vi "Dresden R2R Sputter 03.02.2018 IY24.vi"() -> ()   [LabVIEW 2009] (continued)
                                }
                                }
                                }
                                }
                                frame #1 {
                                }
                                }
                                }
                                }
                              }
                              frame #17 {
                                # "CLOSE PC-BV"
                                n22872 = local read "Yes 4"() -> (w22132:bool)
                                n22873 = case shown="True" w22132 {
                                frame #0 {
                                }
                                frame #1 {
                                n22874 = local read "Semi"() -> (w22133:bool)
                                n22875 = case shown="False" w22133 {
                                frame #0 {
                                n22876 = stacked-sequence {
                                frame #0 {
                                n22877 = local read "Semi"() -> (w22134:bool)
                                n22878 = case shown="False" w22134 {
                                frame #0 {
                                n22879 = stacked-sequence {
                                frame #0 {
                                n22880 = local read "Semi"() -> (w22135:bool)
                                n22881 = case shown="False" w22135 {
                                frame #0 {
                                n22882 = local write "Pc_bv4_auto_close"(TRUE ("Tp1_auto_start")) -> ()
                                }
                                frame #1 {
                                }
                                }
                                }
                                frame #1 {
                                n22883 = local read "Semi"() -> (w22137:bool)
                                n22884 = case shown="False" w22137 {
                                frame #0 {
                                n22885 = Wait (ms)(milliseconds to wait=u32 1000) -> ()  [unwired: 1 out]
                                }
                                frame #1 {
                                }
                                }
                                }
                                frame #2 {
                                n22886 = local read "Semi"() -> (w22139:bool)
                                n22887 = case shown="False" w22139 {
                                frame #0 {
                                n22888 = while {
                                i -> [w22145]
                                stop <- w22141 stop-if-true
                                n22889 = local read "Pc_bv_closed_ch4"() -> (w22143:bool)
                                n22890 = Greater?(x=w22145, y=120) -> (0:w22144:bool)
                                n22891 = local read "Semi"() -> (w22142:bool)
                                n22892 = Compound Arithmetic op=OR(w22142, w22143, w22144) -> (w22141:bool)
                                n22893 = Wait (ms)(milliseconds to wait=u32 500) -> ()  [unwired: 1 out]
                                }
                                }
                                frame #1 {
                                }
                                }
                                }
                                frame #3 {
                                n22894 = local read "Semi"() -> (w22147:bool)
                                n22895 = case shown="False" w22147 {
                                frame #0 {
                                n22896 = local read "Pc_bv_closed_ch4"() -> (w22148:bool)
                                n22897 = case shown="False" w22148 {
                                frame #0 {
                                n22898 = local write "Pc_bv4_auto_close"(TRUE ("Pc_bv1_auto_open")) -> ()
                                }
                                frame #1 {
                                }
                                }
                                }
                                frame #1 {
                                }
                                }
                                }
                                frame #4 {
                                n22899 = local read "Semi"() -> (w22150:bool)
                                n22900 = case shown="False" w22150 {
                                frame #0 {
                                n22901 = local read "Pc_bv_closed_ch1"() -> (w22151:bool)
                                n22902 = case shown="False" w22151 {
                                frame #0 {
                                n22903 = Wait (ms)(milliseconds to wait=u32 1000) -> ()  [unwired: 1 out]
                                }
                                frame #1 {
                                }
                                }
                                }
                                frame #1 {
                                }
                                }
                                }
                                frame #5 {
                                n22904 = local read "Semi"() -> (w22153:bool)
                                n22905 = case shown="False" w22153 {
                                frame #0 {
                                n22906 = while {
                                i -> [w22159]
                                stop <- w22155 stop-if-true
                                n22907 = local read "Pc_bv_closed_ch4"() -> (w22157:bool)
                                n22908 = Greater?(x=w22159, y=120) -> (0:w22158:bool)
                                n22909 = local read "Semi"() -> (w22156:bool)
                                n22910 = Compound Arithmetic op=OR(w22156, w22157, w22158) -> (w22155:bool)
                                n22911 = Wait (ms)(milliseconds to wait=u32 500) -> ()  [unwired: 1 out]
                                }
                                }
                                frame #1 {
                                }
                                }
                                }
                                frame #6 {
                                n22912 = local read "Semi"() -> (w22161:bool)
                                n22913 = case shown="False" w22161 {
                                frame #0 {
                                n22914 = local read "Pc_bv_closed_ch4"() -> (w22162:bool)
                                n22915 = case shown="False" w22162 {
                                frame #0 {
                                n22916 = local write "Error Message"("Shut Down process  cancelled\nbecause  PC-BV not closed.\nPlease check PC-BV4 connections." ("Error Message")) -> ()
                                n22917 = Wait (ms)(milliseconds to wait=u32 1000) -> ()  [unwired: 1 out]
                                }
                                frame #1 {
                                }
                                }
                                }
                                frame #1 {
                                }
                                }
                                }
                                }
                                }
                                frame #1 {
                                }
                                }
                                }
                                frame #1 {
                                n22918 = local read "Semi"() -> (w22165:bool)
                                n22919 = case shown="False" w22165 {
                                frame #0 {
                                n22920 = Wait (ms)(milliseconds to wait=u32 1000) -> ()  [unwired: 1 out]
                                n22921 = local write "Ch4_Sd18"(TRUE ("Ch1_Sd14")) -> ()
                                }
                                frame #1 {
                                }
                                }
                                }
                                }
                                }
                                frame #1 {
                                }
                                }
                                }
                                }
                              }
                              frame #18 {
                                # "CH-VBV CLOSE &  CHECK"
                                n22922 = local read "Semi"() -> (w22168:bool)
                                n22923 = case shown="False" w22168 {
                                frame #0 {
                                n22924 = stacked-sequence {
                                frame #0 {
                                n22925 = local read "Semi"() -> (w22169:bool)
                                n22926 = case shown="False" w22169 {
                                frame #0 {
                                n22927 = while {
                                i -> [w22175]
                                stop <- w22171 stop-if-true
                                n22928 = Greater?(x=w22175, y=50) -> (0:w22174:bool)
                                n22929 = case shown="True" w22174 {
                                frame #0 {
                                }
                                frame #1 {
                                n22930 = local write "Error Message"("Shut Down Process  cancelled\nbecause  CH-VBV  not closed.\nPlease check CH-VBV4 connections." ("Error Message")) -> ()
                                n22931 = local write "Semi"(TRUE ("Semi")) -> ()
                                }
                                }
                                n22932 = local read "Ch4_Ch_vbv_di"() -> (w22170:bool)
                                n22933 = case shown="True" w22170 {
                                tunnel: [TRUE FALSE] -> w22172
                                frame #0 {
                                }
                                frame #1 {
                                n22934 = Wait Until Next ms Multiple(millisecond multiple=u32 500) -> ()  [unwired: 1 out]
                                n22935 = local write "Ch4_Ch_vbv_do"(FALSE ("Ch1_Ch_cc_on_off_di")) -> ()
                                }
                                }
                                n22936 = local read "Semi"() -> (w22173:bool)
                                n22937 = Or(x=w22172, y=w22173) -> (x .or. y?=w22171:bool)
                                }
                                }
                                frame #1 {
                                }
                                }
                                }
                                frame #1 {
                                n22938 = local read "Semi"() -> (w22183:bool)
                                n22939 = case shown="False" w22183 {
                                frame #0 {
                                n22940 = local write "Ch4_Sd19"(TRUE ("Ch1_Sd10 3")) -> ()
                                n22941 = Wait (ms)(milliseconds to wait=u32 1000) -> ()  [unwired: 1 out]
                                }
                                frame #1 {
                                }
                                }
                                }
                                }
                                }
                                frame #1 {
                                }
                                }
                              }
                              frame #19 {
                                # "FINISH SHUTDOWN"
                                n22942 = local read "Semi"() -> (w22186:bool)
                                n22943 = case shown="False" w22186 {
                                frame #0 {
                                n22944 = stacked-sequence {
                                frame #0 {
                                n22945 = local read "Semi"() -> (w22187:bool)
                                n22946 = case shown="False" w22187 {
                                frame #0 {
                                w22188 = TRUE ("Visible")
                                n22947 = property on="final_mes_tab" class="TabCtl (strict)"("Visible"=w22188) -> ()  [unwired: 2 in, 2 out]
                                n22948 = local write "Cnt_Do_Buzzer"(w22188) -> ()
                                n22949 = local write "system_status"("Shut Down Process was completed." ("system_status")) -> ()
                                n22950 = Wait (ms)(milliseconds to wait=u32 3000) -> ()  [unwired: 1 out]
                                }
                                frame #1 {
                                }
                                }
                                }
                                frame #1 {
                                n22951 = local read "Semi"() -> (w22191:bool)
                                n22952 = case shown="False" w22191 {
                                frame #0 {
                                w22192 = FALSE ("Visible")
                                n22953 = property on="final_mes_tab" class="TabCtl (strict)"("Visible"=w22192) -> ()  [unwired: 2 in, 2 out]
                                n22954 = local write "Shutdown_ch4"(w22192) -> ()
                                n22955 = local write "Cnt_Do_Buzzer"(w22192) -> ()
                                n22956 = local write "system_status"("" ("system_status")) -> ()
                                n22957 = Wait (ms)(milliseconds to wait=u32 3000) -> ()  [unwired: 1 out]
                                }
                                frame #1 {
                                }
                                }
                                }
                                frame #2 {
                                n22958 = local read "Semi"() -> (w22195:bool)
                                n22959 = case shown="False" w22195 {
                                frame #0 {
                                n22960 = stacked-sequence {
                                frame #0 {
                                n22961 = local write "Pps_code_entry"("PF233=" ("Pps_code_entry")) -> ()
                                }
                                frame #1 {
                                n22962 = Wait (ms)(milliseconds to wait=u32 500) -> ()  [unwired: 1 out]
                                }
                                frame #2 {
                                n22963 = local write "Ppsok"(TRUE ("Ppsok")) -> ()
                                }
                                frame #3 {
                                n22964 = Wait (ms)(milliseconds to wait=u32 500) -> ()  [unwired: 1 out]
                                }
                                }
                                }
                                frame #1 {
                                }
                                }
                                }
                                frame #3 {
                                n22965 = local read "Semi"() -> (w22200:bool)
                                n22966 = case shown="False" w22200 {
                                frame #0 {
                                n22967 = stacked-sequence {
                                frame #0 {
                                n22968 = local write "Pps_code_entry"("PF234=" ("Pps_code_entry")) -> ()
                                }
                                frame #1 {
                                n22969 = Wait (ms)(milliseconds to wait=u32 500) -> ()  [unwired: 1 out]
                                }
                                frame #2 {
                                n22970 = local write "Ppsok"(TRUE ("Ppsok")) -> ()
                                }
                                frame #3 {
                                n22971 = Wait (ms)(milliseconds to wait=u32 500) -> ()  [unwired: 1 out]
                                }
                                }
                                }
                                frame #1 {
                                }
                                }
                                }
                                frame #4 {
                                n22972 = local read "Semi"() -> (w22205:bool)
                                n22973 = case shown="False" w22205 {
                                frame #0 {
                                n22974 = local write "Ch4_Sd20"(TRUE ("Ch1_Sd15")) -> ()
                                n22975 = Wait (ms)(milliseconds to wait=u32 500) -> ()  [unwired: 1 out]
                                }
                                frame #1 {
                                }
                                }
                                }
                                }
                                }
                                frame #1 {
                                }
                                }
                              }
                            }
                          }
                        }
                      }
                    }
                  }
                  frame #1 {
                  }
                }
              }
            }
          }
          frame #1 {
          }
        }
      }
    }
  }
  n22976 = call <vilib>:"MB Serial Init.vi"("Timeout"=i32? 2000, "Mode"=w792, "Parity"=w794, "Baud Rate"=i32? 9600, "VISA resource name"="Moxa I/O Ch4 Ai") -> ("error out"=w790:errorcluster, "VISA resource name out"=w791:refnum<visa-resource-name>)  [unwired: 2 in, 3 out]
  n22977 = while {
    tunnel: w791 -> [w28291]
    tunnel: w790 -> [w28290]
    tunnel: [w28289] -> w789
    tunnel: [w28288] -> w788
    stop <- FALSE stop-if-true
    n22978 = Wait Until Next ms Multiple(millisecond multiple=u32 300) -> ()  [unwired: 1 out]
    n22979 = stacked-sequence {
      tunnel: [w28297] -> w28289
      tunnel: [w28296] -> w28288
      tunnel: w28291 -> [w28295]
      tunnel: w28290 -> [w28294]
      frame #0 {
        n22980 = local read "Ch4_Ai_CH_PG"() -> (w28303:u16)
        n22981 = local read "Ch4_Ai_CH-CC"() -> (w28300:u16)
        n22982 = local read "1bit="() -> (w28301:dbl)
        n22983 = local read "1bit="() -> (w28304:dbl)
        n22984 = Multiply(x=w28301, y=w28300) -> (x*y=w28299:dbl)
        n22985 = Multiply(x=w28304, y=w28303) -> (x*y=w28302:dbl)
        n22986 = stacked-sequence {
          tunnel: w28302 -> [w28333]
          frame #0 {
            # "CH-PG 0-10 Volt okuma"
            n22987 = feedback #406() -> (w28344:dbl)  [unwired: 1 in]
            n22988 = feedback #407() -> (w28342:dbl)  [unwired: 1 in]
            n22989 = feedback #408() -> (w28341:dbl)  [unwired: 1 in]
            n22990 = feedback #409() -> (w28340:dbl)  [unwired: 1 in]
            n22991 = feedback #410() -> (w28339:dbl)  [unwired: 1 in]
            n22992 = feedback #411() -> (w28338:dbl)  [unwired: 1 in]
            n22993 = feedback #412() -> (w28337:dbl)  [unwired: 1 in]
            n22994 = feedback #413() -> (w28335:dbl)  [unwired: 1 in]
            n22995 = feedback #414() -> (w28336:dbl)  [unwired: 1 in]
            n22996 = Compound Arithmetic op=ADD(w28333, w28344, w28342, w28341, w28340, w28339, w28338, w28337, w28335, w28336) -> (w28343:dbl)
            n22997 = local read "Ch_pg_volt_instantaneous_ch4"() -> (w28326:u16)
            n22998 = Divide(x=w28343, y=u16 10) -> (x/y=w28327:dbl)
            "Ch_pg_volt_ch4" <- w28327
            n22999 = Greater Or Equal?(x=w28326, y=u16 1) -> (x >= y?=w28328:bool)
            n23000 = feedback #415() -> (w28331:bool)  [unwired: 1 in]
            n23001 = case shown="True" w28328 {
              tunnel: w28327 -> [_ w28356]
              tunnel: [FALSE TRUE] -> w28330
              tunnel: w28331 -> [w28347 _]
              tunnel: [w28346 FALSE ("Bg_gui")] -> w28332
              frame #0 {
                n23002 = call "Elapsed Time144"("Reset"=w28347) -> ("Elapsed Time (s)"=w28350:dbl)  [unwired: 11 in, 7 out]
                n23003 = Greater Or Equal?(x=w28350, y=3.0) -> (x >= y?=w28346:bool)
                n23004 = local write "Ch4_Ch_pg_on"(FALSE ("Bg_gui")) -> ()
              }
              frame #1 {
                n23005 = Subtract(x=w28356, y=5.625) -> (x-y=w28358:dbl)
                n23006 = Power Of 10(x=w28358) -> (10^x=w28357:dbl)
                n23007 = In Range and Coerce(upper limit=760.0, x=w28357, lower limit=5e-09) -> (coerced(x)=→"Ch_pg_press_ch4" →"Ch_pg_press_ch4_gui":dbl)  [unwired: 1 out]
                n23008 = local write "Ch4_Ch_pg_on"(TRUE ("Bg_gui")) -> ()
              }
            }
            n23009 = local write "Ch4_Ch_pg_fail"(w28332) -> ()
            "Ch_pg_volt_instantaneous_ch4" <- w28333
          }
        }
        n23010 = stacked-sequence {
          tunnel: w28299 -> [w28415]
          frame #0 {
            # "CH-CC 0-10 Volt okuma"
            n23011 = feedback #416() -> (w28416:dbl)  [unwired: 1 in]
            n23012 = feedback #417() -> (w28417:dbl)  [unwired: 1 in]
            n23013 = feedback #418() -> (w28418:dbl)  [unwired: 1 in]
            n23014 = feedback #419() -> (w28419:dbl)  [unwired: 1 in]
            n23015 = feedback #420() -> (w28420:dbl)  [unwired: 1 in]
            n23016 = feedback #421() -> (w28421:dbl)  [unwired: 1 in]
            n23017 = feedback #422() -> (w28422:dbl)  [unwired: 1 in]
            n23018 = feedback #423() -> (w28434:dbl)  [unwired: 1 in]
            n23019 = feedback #424() -> (w28423:dbl)  [unwired: 1 in]
            n23020 = feedback #425() -> (w28424:dbl)  [unwired: 1 in]
            n23021 = feedback #426() -> (w28425:dbl)  [unwired: 1 in]
            n23022 = feedback #427() -> (w28426:dbl)  [unwired: 1 in]
            n23023 = feedback #428() -> (w28427:dbl)  [unwired: 1 in]
            n23024 = feedback #429() -> (w28428:dbl)  [unwired: 1 in]
            n23025 = feedback #430() -> (w28429:dbl)  [unwired: 1 in]
            n23026 = feedback #431() -> (w28430:dbl)  [unwired: 1 in]
            n23027 = feedback #432() -> (w28431:dbl)  [unwired: 1 in]
            n23028 = feedback #433() -> (w28432:dbl)  [unwired: 1 in]
            n23029 = feedback #434() -> (w28433:dbl)  [unwired: 1 in]
            n23030 = Compound Arithmetic op=ADD(w28415, w28416, w28417, w28418, w28419, w28420, w28421, w28422, w28434, w28423, w28424, w28425, w28426, w28427, w28428, w28429, w28430, w28431, w28432, w28433) -> (w28414:dbl)
            n23031 = Divide(x=w28414, y=u16 20) -> (x/y=w28410:dbl)
            "Ch_CC_volt ch4" <- w28410
            n23032 = feedback #435() -> (w28407:bool)  [unwired: 1 in]
            n23033 = Greater?(x=w28410, y=1.0) -> (0:w28411:bool)
            n23034 = case shown="True" w28411 {
              tunnel: w28410 -> [_ w28449]
              tunnel: [w28442 FALSE] -> w28409
              tunnel: [FALSE ("Ch_cc_on(ch1)") TRUE] -> w28408
              tunnel: w28407 -> [_ _]
              frame #0 {
                n23035 = local read "Ch4_Cc_on_off_di"() -> (w28436:bool)
                n23036 = call "Elapsed Time93"() -> ("Elapsed Time (s)"=w28445:dbl)  [unwired: 12 in, 7 out]
                n23037 = Not(x=w28436) -> (.not. x?=w28439:bool)
                n23038 = Greater Or Equal?(x=w28445, y=3.0) -> (x >= y?=w28444:bool)
                n23039 = call "Elapsed Time94"("Reset"=w28439) -> ("Elapsed Time (s)"=w28441:dbl)  [unwired: 11 in, 7 out]
                n23040 = Greater Or Equal?(x=w28441, y=3.0) -> (x >= y?=w28438:bool)
                n23041 = local write "Ch4_Ch_cc_on"(FALSE ("Ch_cc_on(ch1)")) -> ()
                n23042 = And(x=w28444, y=w28438) -> (x .and. y?=w28442:bool)
              }
              frame #1 {
                n23043 = Subtract(x=w28449, y=10.625) -> (x-y=w28450:dbl)
                n23044 = Power Of X(1:10.0 ("x"), 2:w28450) -> (0:w28455:dbl)
                n23045 = In Range and Coerce(upper limit=1000.0, x=w28455, lower limit=1e-12) -> (coerced(x)=→"Ch_CC_press_ch4" →"Ch_CC_press_ch4_2":dbl)  [unwired: 1 out]
              }
            }
            n23046 = local write "Ch4_Ch_cc_fail"(w28409) -> ()
          }
        }
        n23047 = call-poly <vilib>:"MB Serial Master Query (poly).vi"("VISA resource name"=w28295, "Starting Address"=u16 0, "Quantity"=u16 8, "error in"=w28294, "Serial Parameters"=T39 {"Mode"=enum."RTU", "Slave Address"=1}) -> ("VISA resource name out"=w28297:refnum<visa-resource-name>, "Input Registers"=w28315:u16[], "error out"=w28296:errorcluster)  [unwired: 1 in, 11 out]
        n23048 = Index Array(array=w28315, index=5) -> (element=→"Ch1_Ai_1_5 4":u16)
        n23049 = Index Array(array=w28315, index=6) -> (element=→"Ch1_Ai_1_6 4":u16)
        n23050 = Index Array(array=w28315, index=7) -> (element=→"Ch1_Ai_1_7 4":u16)
        n23051 = Index Array(array=w28315, index=0) -> (element=w28306:u16)
        "Ch4_Ai_PL_PG" <- w28306
        n23052 = Index Array(array=w28315, index=1) -> (element=→"Ch4_Ai_CH_PG":u16)
        n23053 = Index Array(array=w28315, index=2) -> (element=→"Ch4_Ai_CH-CC":u16)
        n23054 = Index Array(array=w28315, index=3) -> (element=→"Ch1_Ai_1_3 4":u16)
        n23055 = Index Array(array=w28315, index=4) -> (element=→"Ch1_Ai_1_4 4":u16)
        n23056 = local read "1bit="() -> (w28307:dbl)
        n23057 = Multiply(x=w28307, y=w28306) -> (x*y=w28305:dbl)
        n23058 = stacked-sequence {
          tunnel: w28305 -> [w28369]
          frame #0 {
            # "PL-PG 0-10 Volt okuma"
            n23059 = feedback #436() -> (w28361:dbl)  [unwired: 1 in]
            n23060 = feedback #437() -> (w28378:dbl)  [unwired: 1 in]
            n23061 = feedback #438() -> (w28377:dbl)  [unwired: 1 in]
            n23062 = feedback #439() -> (w28376:dbl)  [unwired: 1 in]
            n23063 = feedback #440() -> (w28375:dbl)  [unwired: 1 in]
            n23064 = feedback #441() -> (w28374:dbl)  [unwired: 1 in]
            n23065 = feedback #442() -> (w28373:dbl)  [unwired: 1 in]
            n23066 = feedback #443() -> (w28371:dbl)  [unwired: 1 in]
            n23067 = feedback #444() -> (w28372:dbl)  [unwired: 1 in]
            n23068 = Compound Arithmetic op=ADD(w28369, w28361, w28378, w28377, w28376, w28375, w28374, w28373, w28371, w28372) -> (w28379:dbl)
            n23069 = Divide(x=w28379, y=10.0) -> (x/y=w28368:dbl)
            "Pl_pg_volt_ch4" <- w28368
            n23070 = local read "Pl_pg_volt_instantaneous_ch4"() -> (w28367:u16)
            n23071 = Greater Or Equal?(x=w28367, y=u16 1) -> (x >= y?=w28366:bool)
            n23072 = feedback #445() -> (w28363:bool)  [unwired: 1 in]
            n23073 = case shown="True" w28366 {
              tunnel: w28368 -> [_ w28391]
              tunnel: [FALSE TRUE] -> w28364
              tunnel: w28363 -> [w28382 _]
              tunnel: [w28381 FALSE ("Bg_gui")] -> w28362
              frame #0 {
                n23074 = call "Elapsed Time92"("Reset"=w28382) -> ("Elapsed Time (s)"=w28385:dbl)  [unwired: 11 in, 7 out]
                n23075 = local write "Ch4_Pl_pg_on"(FALSE ("Bg_gui")) -> ()
                n23076 = Greater Or Equal?(x=w28385, y=3.0) -> (x >= y?=w28381:bool)
              }
              frame #1 {
                n23077 = Subtract(x=w28391, y=5.625) -> (x-y=w28393:dbl)
                n23078 = Power Of 10(x=w28393) -> (10^x=w28392:dbl)
                n23079 = In Range and Coerce(upper limit=760.0, x=w28392, lower limit=5e-09) -> (coerced(x)=→"Pl_pg_press_ch4" →"Pl_pg_press_ch4_gui":dbl)  [unwired: 1 out]
                n23080 = local write "Ch4_Pl_pg_on"(TRUE ("Bg_gui")) -> ()
              }
            }
            n23081 = local write "Ch4_Pl_pg_fail"(w28362) -> ()
            "Pl_pg_volt_instantaneous_ch4" <- w28369
          }
        }
        n23082 = stacked-sequence {
          frame #0 {
            n23083 = local read "Ch4_Cc_on_off_di"() -> (w28396:bool)
            n23084 = case shown="False" w28396 {
              frame #0 {
                n23085 = local read "Ch_pg_press_ch4"() -> (→"Ch4pressure" →"Ch4_pressure2":dbl)
              }
              frame #1 {
                n23086 = local read "Ch_CC_volt ch4"() -> (w28404:u16)
                n23087 = local read "Ch_pg_volt_ch4"() -> (w28402:u16)
                n23088 = Greater?(x=w28404, y=u16 2) -> (0:w28401:bool)
                n23089 = Less?(x=w28402, y=u16 4) -> (x < y?=w28400:bool)
                n23090 = Or(x=w28401, y=w28400) -> (x .or. y?=w28399:bool)
                n23091 = case shown="False" w28399 {
                  frame #0 {
                    n23092 = local read "Ch_pg_press_ch4"() -> (w28405:dbl)
                    n23093 = local write "Ch4_pressure2"(w28405) -> ()
                    n23094 = local write "Ch4pressure"(w28405) -> ()
                  }
                  frame #1 {
                    n23095 = local read "Ch_CC_press_ch4"() -> (w28406:dbl)
                    n23096 = local write "Ch4_pressure2"(w28406) -> ()
                    n23097 = local write "Ch4pressure"(w28406) -> ()
                  }
                }
              }
            }
          }
        }
      }
    }
  }
  n23098 = while {
    stop <- FALSE stop-if-true
    n23099 = Wait Until Next ms Multiple(millisecond multiple=u32 300) -> ()  [unwired: 1 out]
    n23100 = case shown="True" "Routine_check_transfer" {
      frame #0 {
      }
      frame #1 {
        n23101 = local read "Semi"() -> (w28459:bool)
        n23102 = case shown="False" w28459 {
          frame #0 {
            n23103 = stacked-sequence {
              frame #0 {
                n23104 = local write "Routine_check"(TRUE ("Routine_check")) -> ()
              }
              frame #1 {
                # "SRV-PIST-BACK-CH1"
                n23105 = local read "Semi"() -> (w28461:bool)
                n23106 = case shown="False" w28461 {
                  frame #0 {
                    n23107 = stacked-sequence {
                      frame #0 {
                        n23108 = local read "Semi"() -> (w28462:bool)
                        n23109 = case shown="False" w28462 {
                          frame #0 {
                            n23110 = local write "Ch1_SRV1_PIST For_do"(FALSE ("Ch1_pet_cool_up_do")) -> ()
                          }
                          frame #1 {
                          }
                        }
                      }
                      frame #1 {
                        n23111 = local read "Semi"() -> (w28464:bool)
                        n23112 = case shown="False" w28464 {
                          frame #0 {
                            n23113 = while {
                              i -> [w28470]
                              stop <- w28465 stop-if-true
                              n23114 = Greater?(x=w28470, y=200) -> (0:w28469:bool)
                              n23115 = case shown="True" w28469 {
                                frame #0 {
                                }
                                frame #1 {
                                n23116 = local write "Error Message"("" ("Error Message")) -> ()
                                n23117 = local write "Semi"(TRUE ("Semi")) -> ()
                                }
                              }
                              n23118 = local read "Ch1_SRV1_PIST_Back_di"() -> (w28468:bool)
                              n23119 = case shown="False" w28468 {
                                tunnel: [FALSE TRUE] -> w28467
                                frame #0 {
                                n23120 = local write "Ch1_SRV1_PIST_Back_do"(TRUE ("Ch1_pet_cool_up_do")) -> ()
                                n23121 = Wait Until Next ms Multiple(millisecond multiple=u32 200) -> ()  [unwired: 1 out]
                                }
                                frame #1 {
                                }
                              }
                              n23122 = local read "Semi"() -> (w28466:bool)
                              n23123 = Or(x=w28467, y=w28466) -> (x .or. y?=w28465:bool)
                            }
                          }
                          frame #1 {
                          }
                        }
                      }
                      frame #2 {
                        n23124 = local read "Semi"() -> (w28478:bool)
                        n23125 = case shown="False" w28478 {
                          frame #0 {
                            n23126 = Wait (ms)(milliseconds to wait=u32 200 ("millisecond multiple")) -> ()  [unwired: 1 out]
                            n23127 = local write "RC_1"(TRUE ("RC_1")) -> ()
                          }
                          frame #1 {
                          }
                        }
                      }
                    }
                  }
                  frame #1 {
                  }
                }
              }
              frame #2 {
                # "SRV-PIST-BACK-CH2"
                n23128 = local read "Semi"() -> (w28481:bool)
                n23129 = case shown="False" w28481 {
                  frame #0 {
                    n23130 = stacked-sequence {
                      frame #0 {
                        n23131 = local read "Semi"() -> (w28482:bool)
                        n23132 = case shown="False" w28482 {
                          frame #0 {
                            n23133 = local write "Ch2_SRV1_PIST For_do"(FALSE ("Ch1_pet_cool_up_do")) -> ()
                          }
                          frame #1 {
                          }
                        }
                      }
                      frame #1 {
                        n23134 = local read "Semi"() -> (w28484:bool)
                        n23135 = case shown="False" w28484 {
                          frame #0 {
                            n23136 = while {
                              i -> [w28490]
                              stop <- w28485 stop-if-true
                              n23137 = Greater?(x=w28490, y=200) -> (0:w28489:bool)
                              n23138 = case shown="True" w28489 {
                                frame #0 {
                                }
                                frame #1 {
                                n23139 = local write "Error Message"("" ("Error Message")) -> ()
                                n23140 = local write "Semi"(TRUE ("Semi")) -> ()
                                }
                              }
                              n23141 = local read "Ch2_SRV1_PIST_Back_di"() -> (w28488:bool)
                              n23142 = case shown="False" w28488 {
                                tunnel: [FALSE TRUE] -> w28487
                                frame #0 {
                                n23143 = Wait Until Next ms Multiple(millisecond multiple=u32 200) -> ()  [unwired: 1 out]
                                n23144 = local write "Ch2_SRV1_PIST_Back_do"(TRUE ("Ch1_pet_cool_up_do")) -> ()
                                }
                                frame #1 {
                                }
                              }
                              n23145 = local read "Semi"() -> (w28486:bool)
                              n23146 = Or(x=w28487, y=w28486) -> (x .or. y?=w28485:bool)
                            }
                          }
                          frame #1 {
                          }
                        }
                      }
                      frame #2 {
                        n23147 = local read "Semi"() -> (w28498:bool)
                        n23148 = case shown="False" w28498 {
                          frame #0 {
                            n23149 = local write "RC_2"(TRUE ("RC_2")) -> ()
                            n23150 = Wait (ms)(milliseconds to wait=u32 200 ("millisecond multiple")) -> ()  [unwired: 1 out]
                          }
                          frame #1 {
                          }
                        }
                      }
                    }
                  }
                  frame #1 {
                  }
                }
              }
              frame #3 {
                # "SRV-PIST-BACK-CH3"
                n23151 = local read "Semi"() -> (w28501:bool)
                n23152 = case shown="False" w28501 {
                  frame #0 {
                    n23153 = stacked-sequence {
                      frame #0 {
                        n23154 = local read "Semi"() -> (w28502:bool)
                        n23155 = case shown="False" w28502 {
                          frame #0 {
                            n23156 = local write "Ch3_SRV1_PIST For_do"(FALSE ("Ch1_pet_cool_up_do")) -> ()
                          }
                          frame #1 {
                          }
                        }
                      }
                      frame #1 {
                        n23157 = local read "Semi"() -> (w28504:bool)
                        n23158 = case shown="False" w28504 {
                          frame #0 {
                            n23159 = while {
                              i -> [w28510]
                              stop <- w28505 stop-if-true
                              n23160 = Greater?(x=w28510, y=200) -> (0:w28509:bool)
                              n23161 = case shown="True" w28509 {
                                frame #0 {
                                }
                                frame #1 {
                                n23162 = local write "Error Message"("" ("Error Message")) -> ()
                                n23163 = local write "Semi"(TRUE ("Semi")) -> ()
                                }
                              }
                              n23164 = local read "Ch3_SRV1_PIST_Back_di"() -> (w28508:bool)
                              n23165 = case shown="False" w28508 {
                                tunnel: [FALSE TRUE] -> w28507
                                frame #0 {
                                n23166 = Wait Until Next ms Multiple(millisecond multiple=u32 200) -> ()  [unwired: 1 out]
                                n23167 = local write "Ch3_SRV1_PIST_Back_do"(TRUE ("Ch1_pet_cool_up_do")) -> ()
                                }
                                frame #1 {
                                }
                              }
                              n23168 = local read "Semi"() -> (w28506:bool)
                              n23169 = Or(x=w28507, y=w28506) -> (x .or. y?=w28505:bool)
                            }
                          }
                          frame #1 {
                          }
                        }
                      }
                      frame #2 {
                        n23170 = local read "Semi"() -> (w28518:bool)
                        n23171 = case shown="False" w28518 {
                          frame #0 {
                            n23172 = local write "RC_3"(TRUE ("RC_2")) -> ()
                            n23173 = Wait (ms)(milliseconds to wait=u32 200 ("millisecond multiple")) -> ()  [unwired: 1 out]
                          }
                          frame #1 {
                          }
                        }
                      }
                    }
                  }
                  frame #1 {
                  }
                }
              }
              frame #4 {
                # "SRV-PIST-BACK-CH4"
                n23174 = local read "Semi"() -> (w28521:bool)
                n23175 = case shown="False" w28521 {
                  frame #0 {
                    n23176 = stacked-sequence {
                      frame #0 {
                        n23177 = local read "Semi"() -> (w28522:bool)
                        n23178 = case shown="False" w28522 {
                          frame #0 {
                            n23179 = local write "Ch4_SRV1_PIST For_do"(FALSE ("Ch1_pet_cool_up_do")) -> ()
                          }
                          frame #1 {
                          }
                        }
                      }
                      frame #1 {
                        n23180 = local read "Semi"() -> (w28524:bool)
                        n23181 = case shown="False" w28524 {
                          frame #0 {
                            n23182 = while {
                              i -> [w28530]
                              stop <- w28525 stop-if-true
                              n23183 = Greater?(x=w28530, y=200) -> (0:w28529:bool)
                              n23184 = case shown="True" w28529 {
                                frame #0 {
                                }
                                frame #1 {
                                n23185 = local write "Error Message"("" ("Error Message")) -> ()
                                n23186 = local write "Semi"(TRUE ("Semi")) -> ()
                                }
                              }
                              n23187 = local read "Ch4_SRV1_PIST_Back_di"() -> (w28528:bool)
                              n23188 = case shown="False" w28528 {
                                tunnel: [FALSE TRUE] -> w28527
                                frame #0 {
                                n23189 = Wait Until Next ms Multiple(millisecond multiple=u32 200) -> ()  [unwired: 1 out]
                                n23190 = local write "Ch4_SRV1_PIST_Back_do"(TRUE ("Ch1_pet_cool_up_do")) -> ()
                                }
                                frame #1 {
                                }
                              }
                              n23191 = local read "Semi"() -> (w28526:bool)
                              n23192 = Or(x=w28527, y=w28526) -> (x .or. y?=w28525:bool)
                            }
                          }
                          frame #1 {
                          }
                        }
                      }
                      frame #2 {
                        n23193 = local read "Semi"() -> (w28538:bool)
                        n23194 = case shown="False" w28538 {
                          frame #0 {
                            n23195 = local write "RC_4"(TRUE ("RC_2")) -> ()
                            n23196 = Wait (ms)(milliseconds to wait=u32 200 ("millisecond multiple")) -> ()  [unwired: 1 out]
                          }
                          frame #1 {
                          }
                        }
                      }
                    }
                  }
                  frame #1 {
                  }
                }
              }
              frame #5 {
                # "PET COOL UP-CH1"
                n23197 = local read "Semi"() -> (w28541:bool)
                n23198 = case shown="False" w28541 {
                  frame #0 {
                    n23199 = stacked-sequence {
                      frame #0 {
                        n23200 = local read "Semi"() -> (w28542:bool)
                        n23201 = case shown="False" w28542 {
                          frame #0 {
                            n23202 = local write "Ch1_Pet_cool_down_do"(FALSE ("Ch1_pet_cool_up_do")) -> ()
                          }
                          frame #1 {
                          }
                        }
                      }
                      frame #1 {
                        n23203 = local read "Semi"() -> (w28544:bool)
                        n23204 = case shown="False" w28544 {
                          frame #0 {
                            n23205 = while {
                              i -> [w28550]
                              stop <- w28545 stop-if-true
                              n23206 = Greater?(x=w28550, y=200) -> (0:w28549:bool)
                              n23207 = case shown="True" w28549 {
                                frame #0 {
                                }
                                frame #1 {
                                n23208 = local write "Error Message"("" ("Error Message")) -> ()
                                n23209 = local write "Semi"(TRUE ("Semi")) -> ()
                                }
                              }
                              n23210 = local read "Ch1_Pet_cool_up_di"() -> (w28548:bool)
                              n23211 = case shown="False" w28548 {
                                tunnel: [FALSE TRUE] -> w28547
                                frame #0 {
                                n23212 = Wait Until Next ms Multiple(millisecond multiple=u32 200) -> ()  [unwired: 1 out]
                                n23213 = local write "Ch1_Pet_cool_up_do"(TRUE ("Ch1_pet_cool_up_do")) -> ()
                                }
                                frame #1 {
                                }
                              }
                              n23214 = local read "Semi"() -> (w28546:bool)
                              n23215 = Or(x=w28547, y=w28546) -> (x .or. y?=w28545:bool)
                            }
                          }
                          frame #1 {
                          }
                        }
                      }